vi "Dresden R2R Sputter 03.02.2018 IY24.vi"() -> ()   [LabVIEW 2009] (continued)
          frame #0 {
            # "??????"
            n7666 = Equal To 0?(x=w11957) -> (x = 0?=w11982:bool)
            n7667 = feedback #190() -> (w11979:bool)  [unwired: 1 in]
            n7668 = feedback #191() -> (w11977:bool)  [unwired: 1 in]
            n7669 = Less Or Equal?(x=w11956, y=4500000 ("lower limit")) -> (x <= y?=w11981:bool)
            n7670 = case shown="True" w11982 {
              tunnel: [TRUE FALSE] -> w11980
              tunnel: w11979 -> [_ w12024]
              tunnel: [FALSE w12021] -> w11964
              frame #0 {
              }
              frame #1 {
                n7671 = call "Elapsed Time169"("Reset"=w12024) -> ("Elapsed Time (s)"=w12022:dbl)  [unwired: 11 in, 7 out]
                n7672 = Greater?(x=w12022, y=5.0) -> (0:w12021:bool)
              }
            }
            n7673 = case shown="True" w11981 {
              tunnel: [TRUE FALSE] -> w11978
              tunnel: w11977 -> [_ w12031]
              tunnel: [FALSE w12028] -> w11963
              frame #0 {
              }
              frame #1 {
                n7674 = call "Elapsed Time168"("Reset"=w12031) -> ("Elapsed Time (s)"=w12029:dbl)  [unwired: 11 in, 7 out]
                n7675 = Greater?(x=w12029, y=5.0) -> (0:w12028:bool)
              }
            }
            n7676 = Or(x=w11964, y=w11963) -> (x .or. y?=w11959:bool)
            n7677 = Subtract(x=100.0, y="Warning 1 limit") -> (x-y=w11976:dbl)
            n7678 = Multiply(x=w11976, y=1500000.0) -> (x*y=w11974:dbl)
            n7679 = Divide(x=w11974, y=100.0) -> (x/y=w11971:dbl)
            n7680 = Subtract(x=6000000.0, y=w11971) -> (x-y=w11966:dbl)
            n7681 = feedback #192() -> (w11967:bool)  [unwired: 1 in]
            n7682 = Less Or Equal?(x=w11956, y=w11966) -> (x <= y?=w11968:bool)
            n7683 = case shown="True" w11968 {
              tunnel: [TRUE FALSE] -> w11965
              tunnel: w11967 -> [_ w12017]
              tunnel: [FALSE w12014] -> w11960
              frame #0 {
              }
              frame #1 {
                n7684 = call "Elapsed Time170"("Reset"=w12017) -> ("Elapsed Time (s)"=w12015:dbl)  [unwired: 11 in, 7 out]
                n7685 = Greater?(x=w12015, y=5.0) -> (0:w12014:bool)
              }
            }
            n7686 = case shown="True" w11960 {
              tunnel: [w11988 "Fail" ("Crystal Status :")] -> w11962
              tunnel: [w11987 0.0 ("Crystal Life Time : 2")] -> w11961
              tunnel: w11956 -> [w11986 _]
              tunnel: w11959 -> [w11985 _]
              tunnel: [w11984 TRUE ("Tm1_fail")] -> w11958
              frame #0 {
                n7687 = case shown="True" w11985 {
                  tunnel: ["Good" ("Crystal Status :") "Fail" ("Crystal Status :")] -> w11988
                  tunnel: [w11992 0.0 ("Crystal Life Time : 2")] -> w11987
                  tunnel: w11986 -> [w11991 _]
                  tunnel: [FALSE ("Tm1_fail") TRUE ("Tm1_fail")] -> w11984
                  frame #0 {
                    n7688 = local write "Tm1_Crys_err"(FALSE ("Tm1_Crys_err")) -> ()
                    n7689 = In Range and Coerce(upper limit=6000000, x=w11991, lower limit=4500000) -> (coerced(x)=w12001:u32)  [unwired: 1 out]
                    n7690 = Subtract(x=6000000.0, y=w12001) -> (x-y=w11994:dbl)
                    n7691 = Multiply(x=w11994, y=100.0) -> (x*y=w11996:dbl)
                    n7692 = Divide(x=w11996, y=1500000.0) -> (x/y=w11997:dbl)
                    n7693 = Subtract(x=100.0, y=w11997) -> (x-y=w11992:dbl)
                    "Crystal1_Real" <- w11992
                  }
                  frame #1 {
                    "Tm1_Crys_err" <- TRUE ("Tm1_Cry_err")
                  }
                }
              }
              frame #1 {
                n7694 = local write "Tm1_Crys_err"(TRUE ("Tm1_Crys_err")) -> ()
              }
            }
            "Crystal Status :" <- w11962
            "Crystal Life Time :" <- w11961
            "Crystal Life Time : 2" <- w11961
            n7695 = local write "Tm1_fail"(w11958) -> ()
          }
          frame #1 {
          }
        }
        n7696 = Equal To 0?(x=w11915) -> (x = 0?=w11916:bool)
        n7697 = case shown="False" w11916 {
          tunnel: w11915 -> [w11929 _]
          frame #0 {
            n7698 = Number To Decimal String(number=w11929) -> (decimal integer string=w11931:string)  [unwired: 1 in]
            n7699 = String Subset(string=w11931, offset (0)=0, length (rest)=7 ("length (rest)")) -> (substring=w11930:string)
            n7700 = Decimal String To Number(string=w11930) -> (number=w11923:i32)  [unwired: 2 in, 1 out]
            n7701 = Less?(x=w11923, y=4500000 ("lower limit")) -> (x < y?=w11927:bool)
            n7702 = feedback #193() -> (w11925:bool)  [unwired: 1 in]
            n7703 = case shown="True" w11927 {
              tunnel: [TRUE FALSE] -> w11926
              tunnel: w11925 -> [_ w11953]
              tunnel: [FALSE w11950] -> w11924
              frame #0 {
              }
              frame #1 {
                n7704 = call "Elapsed Time167"("Reset"=w11953) -> ("Elapsed Time (s)"=w11951:dbl)  [unwired: 11 in, 7 out]
                n7705 = Greater?(x=w11951, y=20.0) -> (0:w11950:bool)
              }
            }
            n7706 = case shown="True" w11924 {
              tunnel: w11923 -> [w11934 _]
              frame #0 {
                n7707 = Greater?(x=w11934, y=4500000 ("lower limit")) -> (0:w11937:bool)
                n7708 = Less Or Equal?(x=w11934, y=6000000 ("lower limit")) -> (x <= y?=w11935:bool)
                n7709 = And(x=w11937, y=w11935) -> (x .and. y?=w11936:bool)
                n7710 = case shown="True" w11936 {
                  tunnel: w11934 -> [_ w11940]
                  frame #0 {
                  }
                  frame #1 {
                    n7711 = feedback #194() -> (w11942:i32)  [unwired: 1 in]
                    n7712 = Subtract(x=w11942, y=w11940) -> (x-y=w11944:i32)
                    n7713 = Less?(x=w11944, y=200) -> (x < y?=w11941:bool)
                    n7714 = case shown="True" w11941 {
                      tunnel: w11940 -> [_ w11945]
                      tunnel: w11940 -> [_ _]
                      frame #0 {
                      }
                      frame #1 {
                        "Frequency_short" <- w11945
                      }
                    }
                  }
                }
              }
              frame #1 {
                n7715 = local write "Tm1_fail"(TRUE ("Tm1_fail")) -> ()
                n7716 = local write "Frequency_short"(u32 0 ("Frequency_short")) -> ()
              }
            }
          }
          frame #1 {
            n7717 = local write "Frequency_short"(u32 0 ("Frequency_short")) -> ()
          }
        }
        n7718 = Divide(x=8.83, y="Z_factor") -> (x/y=w11894:dbl)
        n7719 = Subtract(x=w11910, y=w11890) -> (x-y=w11911:dbl)
        n7720 = Divide(x=w11911, y=w11910) -> (x/y=w11909:dbl)
        n7721 = Multiply(x=w11909, y=w11893) -> (x*y=w11908:dbl)
        n7722 = Tangent(1:w11908) -> (0:w11907:dbl)
        n7723 = Multiply(x=w11907, y=w11894) -> (x*y=w11897:dbl)
        n7724 = Inverse Tangent(1:w11897) -> (0:w11896:dbl)
        n7725 = Multiply(x=w11896, y=2.648 ("Pq")) -> (x*y=w11905:dbl)
        n7726 = Multiply(x=w11905, y=166800.0 ("Nq")) -> (x*y=w11903:dbl)
        n7727 = Divide(x=w11903, y=w11893) -> (x/y=w11902:dbl)
        n7728 = Divide(x=w11902, y="Material_density") -> (x/y=w11901:dbl)
        n7729 = Divide(x=w11901, y=w11894) -> (x/y=w11900:dbl)
        n7730 = Divide(x=w11900, y=w11890) -> (x/y=w11898:dbl)
        n7731 = Multiply(x=w11898, y=100000000.0) -> (x*y=w11889:dbl)
        n7732 = Greater?(x=w11889, y=0.0) -> (0:w11891:bool)
        n7733 = case shown="True" w11891 {
          tunnel: w11889 -> [_ w11922]
          frame #0 {
          }
          frame #1 {
            "Snsr_thick" <- w11922
          }
        }
      }
    }
  }
  n7734 = stacked-sequence {
    frame #0 {
      # "TM2"
      n7735 = stacked-sequence {
        tunnel: [_ "Thickness_Monitor2"] -> w12182
        frame #0 {
          n7736 = Wait (ms)(milliseconds to wait=u32 500) -> ()  [unwired: 1 out]
        }
        frame #1 {
        }
      }
      n7737 = call-poly "VISA Configure Serial Port"("VISA resource name"=w12182, "baud rate (9600)"=u32 57600) -> ("VISA resource name out"=w12184:refnum<visa-resource-name>, "error out"=w12183:errorcluster)  [unwired: 12 in]
      n7738 = VISA Clear(VISA resource name=w12184, error in (no error)=w12183) -> (VISA resource name out=w12181:refnum<visa-resource-name>, error out=w12180:errorcluster)
      n7739 = while {
        stop <- FALSE stop-if-true
        n7740 = local read "Tm2_fail"() -> (w12192:bool)
        n7741 = Wait Until Next ms Multiple(millisecond multiple=u32 1000) -> ()  [unwired: 1 out]
        n7742 = case shown="False" w12192 {
          frame #0 {
            # "Rate"
            n7743 = local read "Snsr2_thick"() -> (w12235:dbl)
            n7744 = feedback #195() -> (w12236:dbl)  [unwired: 1 in]
            n7745 = Subtract(x=w12235, y=w12236) -> (x-y=w12216:dbl)
            n7746 = local read "Material_density2"() -> (w12217:dbl)
            n7747 = local read "Z_factor2"() -> (w12218:dbl)
            n7748 = feedback #196() -> (w12232:dbl)  [unwired: 1 in]
            n7749 = feedback #197() -> (w12220:dbl)  [unwired: 1 in]
            n7750 = feedback #198() -> (w12221:dbl)  [unwired: 1 in]
            n7751 = Equal?(x=w12220, y=w12218) -> (x = y?=w12222:bool)
            n7752 = Equal?(x=w12221, y=w12217) -> (x = y?=w12223:bool)
            n7753 = feedback #199() -> (w12231:dbl)  [unwired: 1 in]
            n7754 = And(x=w12222, y=w12223) -> (x .and. y?=w12219:bool)
            n7755 = case shown="True" w12219 {
              tunnel: w12216 -> [_ w12251]
              tunnel: [0.0 w12251] -> w12215
              frame #0 {
                n7756 = Wait (ms)(milliseconds to wait=u32 2000) -> ()  [unwired: 1 out]
              }
              frame #1 {
              }
            }
            n7757 = feedback #200() -> (w12230:dbl)  [unwired: 1 in]
            n7758 = feedback #201() -> (w12229:dbl)  [unwired: 1 in]
            n7759 = feedback #202() -> (w12228:dbl)  [unwired: 1 in]
            n7760 = feedback #203() -> (w12227:dbl)  [unwired: 1 in]
            n7761 = feedback #204() -> (w12226:dbl)  [unwired: 1 in]
            n7762 = feedback #205() -> (w12225:dbl)  [unwired: 1 in]
            n7763 = feedback #206() -> (w12224:dbl)  [unwired: 1 in]
            n7764 = Compound Arithmetic op=ADD(w12215, w12232, w12231, w12230, w12229, w12228, w12227, w12226, w12225, w12224) -> (w12233:dbl)
            n7765 = Divide(x=w12233, y=10.0) -> (x/y=w12212:dbl)
            n7766 = Greater Or Equal?(x=w12212, y=0.0) -> (x >= y?=w12214:bool)
            n7767 = case shown="True" w12214 {
              tunnel: w12212 -> [w12241 _]
              frame #0 {
                # "kA"
                n7768 = Divide(x="Tooling_factor2", y=100.0) -> (x/y=w12242:dbl)
                n7769 = Multiply(x=w12242, y=w12241) -> (x*y=w12237:dbl)
                "Rate2-2" <- w12237
                "Rate2-1" <- w12237
                "Rate2-3" <- w12237
                "Rate2-4" <- w12237
                "Rate 2-5" <- w12237
                n7770 = Divide(x=w12237, y=1000.0) -> (x/y=w12246:dbl)
                n7771 = local read "Thickness 2-1"() -> (w12247:dbl)
                n7772 = Add(x=w12247, y=w12246) -> (x+y=w12239:dbl)
                n7773 = Greater?(x=w12239, y=0.0) -> (0:w12244:bool)
                n7774 = case shown="True" w12244 {
                  tunnel: w12239 -> [_ w12248]
                  frame #0 {
                  }
                  frame #1 {
                    "Thickness 2-1" <- w12248
                    "Thickness 2-2" <- w12248
                    "Thickness 2-3" <- w12248
                  }
                }
              }
              frame #1 {
              }
            }
          }
          frame #1 {
            w12252 = 0.0 ("Rate1-1")
            n7775 = local write "Rate2-1"(w12252) -> ()
            n7776 = local write "Rate2-2"(w12252) -> ()
            n7777 = local write "Rate 2-5"(w12252) -> ()
            n7778 = local write "Rate2-3"(w12252) -> ()
            n7779 = local write "Rate2-4"(w12252) -> ()
          }
        }
        n7780 = Compound Arithmetic op=OR("Tm2_auto_set_zero", "Set2_zero_parameter", "Set2_zero_parameter2") -> (w12188:bool)
        n7781 = case shown="True" w12188 {
          frame #0 {
          }
          frame #1 {
            w12207 = 0.0 ("Thickness 1-1")
            n7782 = local read "Start_coating"() -> (w12202:bool)
            n7783 = local read "Semi"() -> (w12203:bool)
            n7784 = local read "Loading"() -> (w12201:bool)
            n7785 = Compound Arithmetic op=OR(w12203, w12202, w12201) -> (w12204:bool)
            n7786 = case shown="False" w12204 {
              frame #0 {
                n7787 = stacked-sequence {
                  frame #0 {
                    n7788 = local write "Pps_code_entry"("" ("Pps_code_entry")) -> ()
                  }
                  frame #1 {
                    n7789 = Wait (ms)(milliseconds to wait=u32 500) -> ()  [unwired: 1 out]
                  }
                  frame #2 {
                    n7790 = local write "Ppsok"(TRUE ("Ppsok")) -> ()
                  }
                }
              }
              frame #1 {
              }
            }
            n7791 = local write "Set2_zero_parameter2"(FALSE ("Set1_zero_parameter 2")) -> ()
            n7792 = local write "Set2_zero_parameter"(FALSE ("Set1_zero_parameter")) -> ()
            n7793 = local write "Tm2_auto_set_zero"(FALSE ("Tm1_auto_set_zero")) -> ()
            n7794 = local write "Thickness 2-2"(w12207) -> ()
            n7795 = local write "Thickness 2-3"(w12207) -> ()
          }
        }
        n7796 = local read "Frequency_short 2"() -> (w12187:u32)
        n7797 = Not Equal To 0?(x=w12187) -> (x != 0?=w12186:bool)
        n7798 = case shown="True" w12186 {
          frame #0 {
            n7799 = local write "Tm2_gui"(FALSE ("Tm1_fail")) -> ()
          }
          frame #1 {
            n7800 = local read "Thickness 2-1"() -> (w12198:dbl)
            n7801 = Greater?(x=w12198, y="Thickness_for_TM2_gui") -> (0:w12196:bool)
            n7802 = case shown="True" w12196 {
              frame #0 {
                n7803 = local write "Tm2_gui"(FALSE ("Tm1_fail")) -> ()
              }
              frame #1 {
                n7804 = local write "Tm2_gui"(TRUE ("Tm1_fail")) -> ()
              }
            }
          }
        }
      }
      n7805 = while {
        tunnel: w12181 -> [w12405]
        tunnel: w12180 -> [w12404]
        tunnel: [w12398] -> w12179
        tunnel: [w12397] -> w12178
        stop <- FALSE stop-if-true
        n7806 = Wait Until Next ms Multiple(millisecond multiple=u32 250) -> ()  [unwired: 1 out]
        n7807 = case shown="True" "Tm2_set_parameters" {
          frame #0 {
          }
          frame #1 {
            n7808 = stacked-sequence {
              frame #0 {
                n7809 = local write "Pps_code_entry"("" ("Pps_code_entry")) -> ()
              }
              frame #1 {
                n7810 = Wait (ms)(milliseconds to wait=u32 500) -> ()  [unwired: 1 out]
              }
              frame #2 {
                n7811 = local write "Ppsok"(TRUE ("Ppsok")) -> ()
              }
            }
          }
        }
        n7812 = VISA Write(VISA resource name=w12405, write buffer="ª\u0004È¡È\u0001S\u0001\u0000\u0000\u0000Š", error in (no error)=w12404) -> (VISA resource name out=w12407:refnum<visa-resource-name>, error out=w12408:errorcluster)  [unwired: 1 out]
        n7813 = property class="Instr"(reference=w12407, error in=w12408) -> (reference out=w12409:refnum<visa-resource-name>, error out=w12411:errorcluster, "Serial Settings:Number of Bytes at Serial Port"=w12410:u32)
        n7814 = stacked-sequence {
          tunnel: [w12538] -> w12412
          tunnel: w12409 -> [w12538]
          tunnel: [w12537] -> w12414
          tunnel: w12411 -> [w12537]
          tunnel: [w12536] -> w12413
          tunnel: w12410 -> [w12536]
          frame #0 {
            n7815 = Wait (ms)(milliseconds to wait=u32 100) -> ()  [unwired: 1 out]
          }
        }
        n7816 = VISA Read(VISA resource name=w12412, byte count=w12413, error in (no error)=w12414) -> (VISA resource name out=w12398:refnum<visa-resource-name>, read buffer=w12399:string, error out=w12397:errorcluster)  [unwired: 1 out]
        "Tm2_read" <- w12399
        n7817 = String Length(string=w12399) -> (length=w12401:i32)
        n7818 = Greater Or Equal?(x=w12401, y=17) -> (x >= y?=w12400:bool)
        n7819 = case shown="True" w12400 {
          tunnel: w12399 -> [w12418 w12437]
          frame #0 {
            n7820 = String Length(string=w12418) -> (length=w12422:i32)
            n7821 = feedback #207() -> (w12421:bool)  [unwired: 1 in]
            n7822 = Equal To 0?(x=w12422) -> (x = 0?=w12419:bool)
            n7823 = case shown="True" w12419 {
              tunnel: [TRUE FALSE] -> w12420
              tunnel: w12421 -> [_ w12435]
              tunnel: [FALSE w12432] -> w12417
              frame #0 {
              }
              frame #1 {
                n7824 = call "Elapsed Time171"("Reset"=w12435) -> ("Elapsed Time (s)"=w12433:dbl)  [unwired: 11 in, 7 out]
                n7825 = Greater?(x=w12433, y=5.0) -> (0:w12432:bool)
              }
            }
            n7826 = case shown="True" w12417 {
              frame #0 {
                n7827 = local write "Tm2_Conn_err"(FALSE ("TM 1_err")) -> ()
              }
              frame #1 {
                n7828 = local write "Crystal2 Life Time :"(0.0 ("Crystal Life Time :")) -> ()
                n7829 = local write "Oscillator_status 2"(u32 0 ("Oscillator_status")) -> ()
                n7830 = local write "Frequency_long 2"(u32 0 ("Frequency_long")) -> ()
                n7831 = local write "Crystal2 Status :"("") -> ()
                n7832 = local write "Tm2_gui"(FALSE ("Tm1_gui")) -> ()
                "Tm2_Conn_err" <- TRUE ("Tm_Conn_err")
              }
            }
            n7833 = local write "Tm2_fail"(w12417) -> ()
          }
          frame #1 {
            # "hex"
            # "hex"
            # "hex"
            # "hex"
            # "hex"
            n7834 = local write "Tm2_Conn_err"(FALSE ("TM 1_err")) -> ()
            n7835 = Match Pattern(string=w12437, regular expression="ª\t\u0001¡ÈÈS") -> (before substring=w12465:string, after substring=w12466:string)  [unwired: 3 out]
            n7836 = Concatenate Strings(w12466, w12465) -> (w12442:string)
            "Combined_read2" <- w12442
            n7837 = String Subset(string=w12442, offset (0)=4, length (rest)=1 ("length (rest)")) -> (substring=w12443:string)
            n7838 = String Subset(string=w12442, offset (0)=5 ("offset (0) 2"), length (rest)=1 ("length (rest)")) -> (substring=w12444:string)
            n7839 = String Subset(string=w12442, offset (0)=0 ("offset (0) 5"), length (rest)=4 ("length (rest)")) -> (substring=w12459:string)
            n7840 = String Subset(string=w12442, offset (0)=6 ("offset (0) 3"), length (rest)=2 ("length (rest)")) -> (substring=w12445:string)
            n7841 = String Subset(string=w12442, offset (0)=8 ("offset (0) 4"), length (rest)=1 ("length (rest)")) -> (substring=w12446:string)
            n7842 = String To Byte Array(string=w12443) -> (unsigned byte array=w12457:u8[])
            n7843 = String To Byte Array(string=w12445) -> (unsigned byte array=w12451:u8[])
            n7844 = String To Byte Array(string=w12459) -> (unsigned byte array=w12440:u8[])
            n7845 = String To Byte Array(string=w12446) -> (unsigned byte array=w12449:u8[])
            n7846 = String To Byte Array(string=w12444) -> (unsigned byte array=w12455:u8[])
            n7847 = for {
              shift-right: [w12528] -> w12456
              shift-left: "" -> [w12526]
              tunnel: w12457 -> [w12532] mode=indexing
              n7848 = Number To Hexadecimal String(2:w12532) -> (0:w12529:string)  [unwired: 1 in]
              n7849 = String Length(string=w12529) -> (length=w12531:i32)
              n7850 = Less?(x=w12531, y=2) -> (x < y?=w12522:bool)
              n7851 = Select(t="0" ("format string"), s=w12522, f="") -> (s? t:f=w12524:string)
              n7852 = Concatenate Strings(w12524, w12529) -> (w12527:string)
              n7853 = Concatenate Strings(w12526, w12527) -> (w12528:string)
            }
            n7854 = for {
              shift-right: [w12506] -> w12450
              shift-left: "" -> [w12504]
              tunnel: w12451 -> [w12510] mode=indexing
              n7855 = Number To Hexadecimal String(2:w12510) -> (0:w12507:string)  [unwired: 1 in]
              n7856 = String Length(string=w12507) -> (length=w12509:i32)
              n7857 = Less?(x=w12509, y=2) -> (x < y?=w12500:bool)
              n7858 = Select(t="0" ("format string"), s=w12500, f="") -> (s? t:f=w12502:string)
              n7859 = Concatenate Strings(w12502, w12507) -> (w12505:string)
              n7860 = Concatenate Strings(w12504, w12505) -> (w12506:string)
            }
            n7861 = for {
              shift-right: [w12484] -> w12439
              shift-left: "" -> [w12482]
              tunnel: w12440 -> [w12488] mode=indexing
              n7862 = Number To Hexadecimal String(2:w12488) -> (0:w12485:string)  [unwired: 1 in]
              n7863 = String Length(string=w12485) -> (length=w12487:i32)
              n7864 = Less?(x=w12487, y=2) -> (x < y?=w12478:bool)
              n7865 = Select(t="0" ("format string"), s=w12478, f="") -> (s? t:f=w12480:string)
              n7866 = Concatenate Strings(w12480, w12485) -> (w12483:string)
              n7867 = Concatenate Strings(w12482, w12483) -> (w12484:string)
            }
            n7868 = for {
              shift-right: [w12495] -> w12447
              shift-left: "" -> [w12493]
              tunnel: w12449 -> [w12499] mode=indexing
              n7869 = Number To Hexadecimal String(2:w12499) -> (0:w12496:string)  [unwired: 1 in]
              n7870 = String Length(string=w12496) -> (length=w12498:i32)
              n7871 = Less?(x=w12498, y=2) -> (x < y?=w12489:bool)
              n7872 = Select(t="0" ("format string"), s=w12489, f="") -> (s? t:f=w12491:string)
              n7873 = Concatenate Strings(w12491, w12496) -> (w12494:string)
              n7874 = Concatenate Strings(w12493, w12494) -> (w12495:string)
            }
            n7875 = for {
              shift-right: [w12517] -> w12453
              shift-left: "" -> [w12515]
              tunnel: w12455 -> [w12521] mode=indexing
              n7876 = Number To Hexadecimal String(2:w12521) -> (0:w12518:string)  [unwired: 1 in]
              n7877 = String Length(string=w12518) -> (length=w12520:i32)
              n7878 = Less?(x=w12520, y=2) -> (x < y?=w12511:bool)
              n7879 = Select(t="0" ("format string"), s=w12511, f="") -> (s? t:f=w12513:string)
              n7880 = Concatenate Strings(w12513, w12518) -> (w12516:string)
              n7881 = Concatenate Strings(w12515, w12516) -> (w12517:string)
            }
            n7882 = Hexadecimal String To Number(string=w12450) -> (number=→"Measurement_time 2":u32)  [unwired: 2 in, 1 out]
            n7883 = Hexadecimal String To Number(string=w12453) -> (number=→"Sample_number 2":u32)  [unwired: 2 in, 1 out]
            n7884 = Hexadecimal String To Number(string=w12456) -> (number=→"Oscillator_status 2":u32)  [unwired: 2 in, 1 out]
            n7885 = Hexadecimal String To Number(string=w12439) -> (number=→"Frequency_long 2":u32)  [unwired: 2 in, 1 out]
            n7886 = Hexadecimal String To Number(string=w12447) -> (number=→"Device_ID 2":u32)  [unwired: 2 in, 1 out]
          }
        }
      }
      n7887 = VISA Close(VISA resource name=w12179, error in (no error)=w12178) -> ()  [unwired: 1 out]
      n7888 = while {
        stop <- FALSE stop-if-true
        w12274 = 6000000.0 ("Fq")
        w12257 = 3.141592653589793
        # "cm"
        # "Tickness \n    (cm)"
        # "density of quartz \n2.648 g/cm3"
        # "Frequency constants \n1.668 E+5 Hz · cm"
        # "Frequency Of Loaded \nSensor Crystal"
        # "Si02 Acoustic Impedance"
        # "Si02 Acoustic Impedance"
        n7889 = local read "Frequency_short 2"() -> (w12254:u32)
        n7890 = Wait Until Next ms Multiple(millisecond multiple=u32 250) -> ()  [unwired: 1 out]
        n7891 = local read "Tm2_read"() -> (w12282:string)
        n7892 = local read "Oscillator_status 2"() -> (w12276:u32)
        n7893 = local read "Frequency_long 2"() -> (w12279:u32)
        n7894 = Equal?(x=w12282, y="") -> (x = y?=w12281:bool)
        n7895 = case shown="False" w12281 {
          tunnel: w12254 -> [_ _]
          tunnel: w12276 -> [w12321 _]
          tunnel: w12254 -> [w12320 _]
          frame #0 {
            n7896 = Equal To 0?(x=w12321) -> (x = 0?=w12346:bool)
            n7897 = feedback #208() -> (w12343:bool)  [unwired: 1 in]
            n7898 = feedback #209() -> (w12341:bool)  [unwired: 1 in]
            n7899 = Less Or Equal?(x=w12320, y=4500000 ("lower limit")) -> (x <= y?=w12345:bool)
            n7900 = case shown="True" w12346 {
              tunnel: [TRUE FALSE] -> w12344
              tunnel: w12343 -> [_ w12388]
              tunnel: [FALSE w12385] -> w12328
              frame #0 {
              }
              frame #1 {
                n7901 = call "Elapsed Time173"("Reset"=w12388) -> ("Elapsed Time (s)"=w12386:dbl)  [unwired: 11 in, 7 out]
                n7902 = Greater?(x=w12386, y=5.0) -> (0:w12385:bool)
              }
            }
            n7903 = case shown="True" w12345 {
              tunnel: [TRUE FALSE] -> w12342
              tunnel: w12341 -> [_ w12395]
              tunnel: [FALSE w12392] -> w12327
              frame #0 {
              }
              frame #1 {
                n7904 = call "Elapsed Time172"("Reset"=w12395) -> ("Elapsed Time (s)"=w12393:dbl)  [unwired: 11 in, 7 out]
                n7905 = Greater?(x=w12393, y=5.0) -> (0:w12392:bool)
              }
            }
            n7906 = Or(x=w12328, y=w12327) -> (x .or. y?=w12323:bool)
            n7907 = Subtract(x=100.0, y="Warning 2 limit") -> (x-y=w12340:dbl)
            n7908 = Multiply(x=w12340, y=1500000.0) -> (x*y=w12338:dbl)
            n7909 = Divide(x=w12338, y=100.0) -> (x/y=w12335:dbl)
            n7910 = Subtract(x=6000000.0, y=w12335) -> (x-y=w12330:dbl)
            n7911 = feedback #210() -> (w12331:bool)  [unwired: 1 in]
            n7912 = Less Or Equal?(x=w12320, y=w12330) -> (x <= y?=w12332:bool)
            n7913 = case shown="True" w12332 {
              tunnel: [TRUE FALSE] -> w12329
              tunnel: w12331 -> [_ w12381]
              tunnel: [FALSE w12378] -> w12324
              frame #0 {
              }
              frame #1 {
                n7914 = call "Elapsed Time174"("Reset"=w12381) -> ("Elapsed Time (s)"=w12379:dbl)  [unwired: 11 in, 7 out]
                n7915 = Greater?(x=w12379, y=5.0) -> (0:w12378:bool)
              }
            }
            n7916 = case shown="False" w12324 {
              tunnel: [w12352 "Fail" ("Crystal Status :")] -> w12326
              tunnel: [w12351 0.0 ("Crystal Life Time : 2")] -> w12325
              tunnel: w12320 -> [w12350 _]
              tunnel: w12323 -> [w12349 _]
              tunnel: [w12348 TRUE ("Tm1_fail")] -> w12322
              frame #0 {
                n7917 = case shown="True" w12349 {
                  tunnel: ["Good" ("Crystal Status :") "Fail" ("Crystal Status :")] -> w12352
                  tunnel: [w12356 0.0 ("Crystal Life Time : 2")] -> w12351
                  tunnel: w12350 -> [w12355 _]
                  tunnel: [FALSE ("Tm1_fail") TRUE ("Tm1_fail")] -> w12348
                  frame #0 {
                    n7918 = local write "Tm2_Crys_err"(FALSE ("Tm1_Crys_err")) -> ()
                    n7919 = In Range and Coerce(upper limit=6000000, x=w12355, lower limit=4500000) -> (coerced(x)=w12365:u32)  [unwired: 1 out]
                    n7920 = Subtract(x=6000000.0, y=w12365) -> (x-y=w12358:dbl)
                    n7921 = Multiply(x=w12358, y=100.0) -> (x*y=w12360:dbl)
                    n7922 = Divide(x=w12360, y=1500000.0) -> (x/y=w12361:dbl)
                    n7923 = Subtract(x=100.0, y=w12361) -> (x-y=w12356:dbl)
                    "Crystal2_Real" <- w12356
                  }
                  frame #1 {
                    "Tm2_Crys_err" <- TRUE ("Tm1_Cry_err")
                  }
                }
              }
              frame #1 {
                n7924 = local write "Tm2_Crys_err"(TRUE ("Tm1_Crys_err")) -> ()
              }
            }
            "Crystal2 Status :" <- w12326
            "Crystal2 Life Time :" <- w12325
            "Crystal2 Life Time : 2" <- w12325
            n7925 = local write "Tm2_fail"(w12322) -> ()
          }
          frame #1 {
          }
        }
        n7926 = Equal To 0?(x=w12279) -> (x = 0?=w12280:bool)
        n7927 = case shown="False" w12280 {
          tunnel: w12279 -> [w12293 _]
          frame #0 {
            n7928 = Number To Decimal String(number=w12293) -> (decimal integer string=w12295:string)  [unwired: 1 in]
            n7929 = String Subset(string=w12295, offset (0)=0, length (rest)=7 ("length (rest)")) -> (substring=w12294:string)
            n7930 = Decimal String To Number(string=w12294) -> (number=w12287:i32)  [unwired: 2 in, 1 out]
            n7931 = Less?(x=w12287, y=4500000 ("lower limit")) -> (x < y?=w12291:bool)
            n7932 = feedback #211() -> (w12289:bool)  [unwired: 1 in]
            n7933 = case shown="True" w12291 {
              tunnel: [TRUE FALSE] -> w12290
              tunnel: w12289 -> [_ w12317]
              tunnel: [FALSE w12314] -> w12288
              frame #0 {
              }
              frame #1 {
                n7934 = call "Elapsed Time175"("Reset"=w12317) -> ("Elapsed Time (s)"=w12315:dbl)  [unwired: 11 in, 7 out]
                n7935 = Greater?(x=w12315, y=20.0) -> (0:w12314:bool)
              }
            }
            n7936 = case shown="False" w12288 {
              tunnel: w12287 -> [w12298 _]
              frame #0 {
                n7937 = Greater?(x=w12298, y=4500000 ("lower limit")) -> (0:w12301:bool)
                n7938 = Less Or Equal?(x=w12298, y=6000000 ("lower limit")) -> (x <= y?=w12299:bool)
                n7939 = And(x=w12301, y=w12299) -> (x .and. y?=w12300:bool)
                n7940 = case shown="True" w12300 {
                  tunnel: w12298 -> [_ w12304]
                  frame #0 {
                  }
                  frame #1 {
                    n7941 = feedback #212() -> (w12306:i32)  [unwired: 1 in]
                    n7942 = Subtract(x=w12306, y=w12304) -> (x-y=w12308:i32)
                    n7943 = Less?(x=w12308, y=200) -> (x < y?=w12305:bool)
                    n7944 = case shown="True" w12305 {
                      tunnel: w12304 -> [_ w12309]
                      tunnel: w12304 -> [_ _]
                      frame #0 {
                      }
                      frame #1 {
                        "Frequency_short 2" <- w12309
                      }
                    }
                  }
                }
              }
              frame #1 {
                n7945 = local write "Tm2_fail"(TRUE ("Tm1_fail")) -> ()
                n7946 = local write "Frequency_short 2"(u32 0 ("Frequency_short")) -> ()
              }
            }
          }
          frame #1 {
            n7947 = local write "Frequency_short 2"(u32 0 ("Frequency_short")) -> ()
          }
        }
        n7948 = Divide(x=8.83, y="Z_factor2") -> (x/y=w12258:dbl)
        n7949 = Subtract(x=w12274, y=w12254) -> (x-y=w12275:dbl)
        n7950 = Divide(x=w12275, y=w12274) -> (x/y=w12273:dbl)
        n7951 = Multiply(x=w12273, y=w12257) -> (x*y=w12272:dbl)
        n7952 = Tangent(1:w12272) -> (0:w12271:dbl)
        n7953 = Multiply(x=w12271, y=w12258) -> (x*y=w12261:dbl)
        n7954 = Inverse Tangent(1:w12261) -> (0:w12260:dbl)
        n7955 = Multiply(x=w12260, y=2.648 ("Pq")) -> (x*y=w12269:dbl)
        n7956 = Multiply(x=w12269, y=166800.0 ("Nq")) -> (x*y=w12267:dbl)
        n7957 = Divide(x=w12267, y=w12257) -> (x/y=w12266:dbl)
        n7958 = Divide(x=w12266, y="Material_density2") -> (x/y=w12265:dbl)
        n7959 = Divide(x=w12265, y=w12258) -> (x/y=w12264:dbl)
        n7960 = Divide(x=w12264, y=w12254) -> (x/y=w12262:dbl)
        n7961 = Multiply(x=w12262, y=100000000.0) -> (x*y=w12253:dbl)
        n7962 = Greater?(x=w12253, y=0.0) -> (0:w12255:bool)
        n7963 = case shown="True" w12255 {
          tunnel: w12253 -> [_ w12286]
          frame #0 {
          }
          frame #1 {
            "Snsr2_thick" <- w12286
          }
        }
      }
    }
  }
  n7964 = call <vilib>:"MB Serial Init.vi"(10:i32? 115200 ("Baud Rate"), 11:"Merobel Tension Controller 2") -> (0:w736, 3:w737)  [unwired: 8 in]
  n7965 = call <vilib>:"MB Serial Init.vi"("Timeout"=i32? 4000, "Mode"=w780, "Parity"=w778, "Baud Rate"=i32? 9600, "VISA resource name"="Moxa I/O Ch 1") -> ("error out"=w775:errorcluster, "VISA resource name out"=w749:refnum<visa-resource-name>)  [unwired: 2 in, 3 out]
  n7966 = while {
    tunnel: [w12548] -> w758
    tunnel: [w12547] -> w757
    tunnel: w756 -> [w12546]
    tunnel: w755 -> [w12545]
    tunnel: "milliseconds to wait 5" -> [w12542]
    stop <- FALSE stop-if-true
    n7967 = stacked-sequence {
      tunnel: [w12553 _] -> w12548
      tunnel: [w12552 _] -> w12547
      tunnel: w12546 -> [w12551 _]
      tunnel: w12545 -> [w12550 _]
      tunnel: w12542 -> [w12549 _]
      frame #0 {
        n7968 = stacked-sequence {
          tunnel: w12550 -> [w12568 _ _ _ _ _ _ _]
          tunnel: w12551 -> [w12567 _ _ _ _ _ _ _]
          tunnel: [_ _ _ _ _ _ w12732 _] -> w12552
          tunnel: [_ _ _ _ _ _ w12731 _] -> w12553
          tunnel: w12549 -> [_ w12646 _ w12662 _ w12717 _ w12744]
          frame #0 {
            # "Digital I/O & Analog \nOutput Part"
            n7969 = call-poly <vilib>:"MB Serial Master Query (poly).vi"("VISA resource name"=w12568, "Starting Address"=u16 0, "Quantity"=u16 8, "error in"=w12567, "Serial Parameters"=T39 {"Mode"=enum."RTU", "Slave Address"=2}) -> ("VISA resource name out"=w12566:refnum<visa-resource-name>, "Discrete Inputs"=w12635:bool[], "error out"=w12565:errorcluster)  [unwired: 2 in, 10 out]
            n7970 = Index Array(array=w12635, index=7) -> (element=w12629:bool)
            "Ch4_Cc_on_off_di" <- w12629
            n7971 = Index Array(array=w12635, index=5) -> (element=w12558:bool)
            "Ch4_Pl_vbv_di" <- w12558
            n7972 = Index Array(array=w12635, index=6) -> (element=w12630:bool)
            "Ch4_Pl_atm_di" <- w12630
            n7973 = Index Array(array=w12635, index=0) -> (element=w12633:bool)
            "Ch4_Mp_di" <- w12633
            n7974 = Index Array(array=w12635, index=1) -> (element=w12628:bool)
            "Ch4_Tp_bv_di" <- w12628
            n7975 = Index Array(array=w12635, index=2) -> (element=w12632:bool)
            "Ch4_Bg_bv_di" <- w12632
            n7976 = Index Array(array=w12635, index=3) -> (element=w12631:bool)
            "Ch4_Ch_vbv_di" <- w12631
            n7977 = Index Array(array=w12635, index=4) -> (element=w12627:bool)
            "Ch4_Ch_atm_di" <- w12627
            n7978 = local write "Ch4_Ch_vbv_on"(w12631) -> ()
            n7979 = local write "Ch4_Ch_atm_on"(w12627) -> ()
            n7980 = local write "Ch4_Tp_bv_on"(w12628) -> ()
            n7981 = local write "Ch4_Bg_bv_on"(w12632) -> ()
            n7982 = local write "Ch4_Pl_atm_on"(w12630) -> ()
            n7983 = local write "Ch4_Ch_cc_on"(w12629) -> ()
            n7984 = local write "Ch4_Pl_vbv_on"(w12558) -> ()
            n7985 = local write "Ch4_Mp_on"(w12633) -> ()
            n7986 = call-poly <vilib>:"MB Serial Master Query (poly).vi"("VISA resource name"=w12566, "Starting Address"=u16 0, "Quantity"=u16 8, "error in"=w12565, "Serial Parameters"=T39 {"Mode"=enum."RTU", "Slave Address"=3}) -> ("VISA resource name out"=w12564:refnum<visa-resource-name>, "Discrete Inputs"=w12615:bool[], "error out"=w12563:errorcluster)  [unwired: 1 in, 11 out]
            n7987 = local read "Load_dido"() -> (w12557:bool)
            n7988 = case shown="True" w12557 {
              frame #0 {
              }
              frame #1 {
                n7989 = Wait (ms)(milliseconds to wait=u32 2000) -> ()  [unwired: 1 out]
              }
            }
            n7990 = Index Array(array=w12615, index=5) -> (element=w12555:bool)
            "Ch4_Cst_fix_down_di" <- w12555
            n7991 = Index Array(array=w12615, index=6) -> (element=→"Ch4_Pet_cool_up_di":bool)
            n7992 = Index Array(array=w12615, index=7) -> (element=→"Ch4_Pet_cool_down_di":bool)
            n7993 = Index Array(array=w12615, index=0) -> (element=w12556:bool)
            "Ch4_Sov_Ar_di" <- w12556
            n7994 = Index Array(array=w12615, index=1) -> (element=→"Ch4_Di_1_1":bool)
            n7995 = Index Array(array=w12615, index=2) -> (element=→"Ch4_Di_1_2":bool)
            n7996 = Index Array(array=w12615, index=3) -> (element=w12554:bool)
            "Ch4_Trns_gv_bp_di" <- w12554
            n7997 = Index Array(array=w12615, index=4) -> (element=→"Ch4_Cst_fix_up_di":bool)
            n7998 = local write "Trns_gv_bp_ch4_on_top"(w12554) -> ()
            n7999 = local write "Trns_gv_bp_on_ch4_front"(w12554) -> ()
            n8000 = local write "Ch4_Trns_gv_bp_on"(w12554) -> ()
            n8001 = local write "ch4_sov_Ar_on_top"(w12556) -> ()
            n8002 = local write "chamber 4 top piston open"(w12555) -> ()
            n8003 = call-poly <vilib>:"MB Serial Master Query (poly).vi"("VISA resource name"=w12564, "Starting Address"=u16 0, "Quantity"=u16 8, "error in"=w12563, "Serial Parameters"=T39 {"Mode"=enum."RTU", "Slave Address"=4}) -> ("VISA resource name out"=w12562:refnum<visa-resource-name>, "Discrete Inputs"=w12573:bool[], "error out"=w12561:errorcluster)  [unwired: 1 in, 11 out]
            n8004 = Index Array(array=w12573, index=5) -> (element=→"Ch4_SRV2_counter_di":bool)
            n8005 = Index Array(array=w12573, index=6) -> (element=→"Ch4_WFS_di":bool)
            n8006 = Index Array(array=w12573, index=7) -> (element=→"Ch4_4_7_di":bool)
            n8007 = Index Array(array=w12573, index=0) -> (element=→"Ch4_SRV1_PIST For_di":bool)
            n8008 = Index Array(array=w12573, index=1) -> (element=→"Ch4_SRV1_PIST_Back_di":bool)
            n8009 = Index Array(array=w12573, index=2) -> (element=→"Ch4_SRV_start_stop_di":bool)
            n8010 = Index Array(array=w12573, index=3) -> (element=→"Ch4_SRV_left_direction_di":bool)
            n8011 = Index Array(array=w12573, index=4) -> (element=→"Ch4_SRV1_counter_di":bool)
            n8012 = call-poly <vilib>:"MB Serial Master Query (poly).vi"("VISA resource name"=w12562, "Starting Address"=u16 0, "Quantity"=u16 8, "error in"=w12561, "Serial Parameters"=T39 {"Mode"=enum."RTU", "Slave Address"=5}) -> ("VISA resource name out"=w12560:refnum<visa-resource-name>, "Discrete Inputs"=w12593:bool[], "error out"=w12559:errorcluster)  [unwired: 1 in, 11 out]
            n8013 = Index Array(array=w12593, index=5) -> (element=→"Ch4_4_5_di":bool)
            n8014 = Index Array(array=w12593, index=6) -> (element=→"Ch4_Left_slow_di":bool)
            n8015 = Index Array(array=w12593, index=7) -> (element=→"Ch4_Left_limit_di":bool)
            n8016 = Index Array(array=w12593, index=0) -> (element=→"Ch4_Air_press_di":bool)
            n8017 = Index Array(array=w12593, index=1) -> (element=→"Ch4_Ds_di":bool)
            n8018 = Index Array(array=w12593, index=2) -> (element=→"Ch4_TGV_control_di":bool)
            n8019 = Index Array(array=w12593, index=3) -> (element=→"Ch4_Trns_interlock_di":bool)
            n8020 = Index Array(array=w12593, index=4) -> (element=→"Ch4_4_4_di":bool)
          }
          frame #1 {
            n8021 = Wait (ms)(milliseconds to wait=w12646) -> ()  [unwired: 1 out]
          }
          frame #2 {
            n8022 = local read "Load_dido"() -> (w12647:bool)
            n8023 = case shown="True" w12647 {
              frame #0 {
              }
              frame #1 {
                n8024 = while {
                  stop <- w12654 stop-if-true
                  n8025 = local read "Ch4_Cst_fix_down_di"() -> (w12651:bool)
                  n8026 = local read "Ch4_Trns_gv_bp_di"() -> (w12652:bool)
                  n8027 = local read "Ch4_Pet_cool_up_di"() -> (w12650:bool)
                  n8028 = local read "Ch4_Pet_cool_down_di"() -> (w12649:bool)
                  n8029 = local read "Ch4_Mp_di"() -> (w12661:bool)
                  n8030 = local read "Ch4_Tp_bv_di"() -> (w12660:bool)
                  n8031 = local read "Ch4_Bg_bv_di"() -> (w12659:bool)
                  n8032 = local read "Ch4_Ch_vbv_di"() -> (w12658:bool)
                  n8033 = local read "Ch4_Pl_vbv_di"() -> (w12657:bool)
                  n8034 = local read "Ch4_Cc_on_off_di"() -> (w12656:bool)
                  n8035 = local read "Ch4_WFS_di"() -> (w12648:bool)
                  n8036 = local write "Ch4_WFC_do"(w12648) -> ()
                  n8037 = local write "Ch4_Mp_do"(w12661) -> ()
                  n8038 = local write "Ch4_Tp_bv_do"(w12660) -> ()
                  n8039 = local write "Ch4_Bg_bv_do"(w12659) -> ()
                  n8040 = local write "Ch4_Ch_vbv_do"(w12658) -> ()
                  n8041 = local write "Ch4_Pl_vbv_do"(w12657) -> ()
                  n8042 = local write "Ch4_Trns_gv_bp_do"(w12652) -> ()
                  n8043 = local write "Ch4_Pet_cool_up_do"(w12650) -> ()
                  n8044 = local write "Ch4_Pet_cool_down_do"(w12649) -> ()
                  n8045 = local write "Ch4_Cc_on_off_do"(w12656) -> ()
                  n8046 = local write "Ch4_Cst_fix_do"(w12651) -> ()
                  n8047 = local read "Load_dido"() -> (w12655:bool)
                  n8048 = Wait Until Next ms Multiple(millisecond multiple=u32 300) -> ()  [unwired: 1 out]
                  n8049 = Not(x=w12655) -> (.not. x?=w12654:bool)
                }
              }
            }
          }
          frame #3 {
            n8050 = Wait (ms)(milliseconds to wait=w12662) -> ()  [unwired: 1 out]
          }
          frame #4 {
            n8051 = Build Array("Ch4_Mp_do", "Ch4_Tp_bv_do", "Ch4_Bg_bv_do", "Ch4_Ch_vbv_do", "Ch4_Ch_atm_do", "Ch4_Pl_vbv_do", "Ch4_Pl_atm_do", "Ch4_Cc_on_off_do") -> (w12686:bool[])
            n8052 = call-poly <vilib>:"MB Serial Master Query (poly).vi"("VISA resource name"=w12678, "Starting Address"=u16 320, "Coils"=w12686, "error in"=w12677, "Serial Parameters"=T39 {"Mode"=enum."RTU", "Slave Address"=2}) -> ("VISA resource name out"=w12676:refnum<visa-resource-name>, "error out"=w12675:errorcluster)  [unwired: 1 in, 12 out]
            n8053 = Build Array("Ch4_Sov_Ar_do", "Ch4_Do_1_1", "Ch4_Do_1_2", "Ch4_Trns_gv_bp_do", "Ch4_Cst_fix_do", "Ch4_2_5_di", "Ch4_Pet_cool_up_do", "Ch4_Pet_cool_down_do") -> (w12696:bool[])
            n8054 = call-poly <vilib>:"MB Serial Master Query (poly).vi"("VISA resource name"=w12676, "Starting Address"=u16 320, "Coils"=w12696, "error in"=w12675, "Serial Parameters"=T39 {"Mode"=enum."RTU", "Slave Address"=3}) -> ("VISA resource name out"=w12673:refnum<visa-resource-name>, "error out"=w12674:errorcluster)  [unwired: 1 in, 12 out]
            n8055 = Build Array("Ch4_SRV1_PIST For_do", "Ch4_SRV1_PIST_Back_do", "Ch4_SRV_start_stop_do", "Ch4_SRV_counterclockwise_direction_do", "Ch4_Do_3_4", "Ch4_Do_3_5", "Ch4_WFC_do", "Ch4_Do_3_7") -> (w12706:bool[])
            n8056 = call-poly <vilib>:"MB Serial Master Query (poly).vi"("VISA resource name"=w12673, "Starting Address"=u16 320, "Coils"=w12706, "error in"=w12674, "Serial Parameters"=T39 {"Mode"=enum."RTU", "Slave Address"=4}) -> ("VISA resource name out"=w12671:refnum<visa-resource-name>, "error out"=w12672:errorcluster)  [unwired: 1 in, 12 out]
            n8057 = Build Array("Ch4_4_0_do", "Ch4_4_1_do", "Ch4_TGV_control_do", "Ch4_4_3_do", "Ch4_4_4_do", "Ch4_Do_4_5", "Ch4_Do_4_6", "Ch4_Do_4_7") -> (w12716:bool[])
            n8058 = call-poly <vilib>:"MB Serial Master Query (poly).vi"("VISA resource name"=w12671, "Starting Address"=u16 320, "Coils"=w12716, "error in"=w12672, "Serial Parameters"=T39 {"Mode"=enum."RTU", "Slave Address"=5}) -> ("VISA resource name out"=w12670:refnum<visa-resource-name>, "error out"=w12669:errorcluster)  [unwired: 1 in, 12 out]
          }
          frame #5 {
            n8059 = Wait (ms)(milliseconds to wait=w12717) -> ()  [unwired: 1 out]
          }
          frame #6 {
            n8060 = Build Array(FALSE, "Ch4_Ao_1_0", "Ch4_Ao_1_1", "Ch4_Ao_1_2", "Ch4_Ao_1_3") -> (w12724:bool[])